vi "extract galvo voltage readout clusterinput (SubVI).vi"(0 "file path (use dialog)":path=path "F:/20220627-135231calib/waveforms.pico", 5 "cluster":T1={"# of avg for single waveform"=0, "skip [us]"=0.0, "Nzf*Nv"=0, "ofst"=0.0, "# of avg for volumes"=0, "limit data length"=FALSE, "num of frames"=7500, "Nv"=7500}) -> (3 "element":dbl=5713585.0 format="%#.6g", 4 "sampling period [s]":dbl=2.0000000000000002e-07, 6 "img scan tangent":dbl[][](array[numeric]), 8 "path":path=path "F:/20220627-135231calib/waveforms.pico", 10 "img scan voltage":dbl[][](array[numeric]), 14 "img scan monitor":dbl[][](array[numeric])=[[17426.8575, 17426.57890625, 17426.393014705885, 17426.015972222223, 17426.046052631584, 17426.081875000003, 17426.223214285717, 17426.462215909094, 17426.573641304352, 17426.58333333334, 17426.650000000005, 17426.70192307693, 17426.684259259262, 17426.62790178572, 17426.683405172418, 17426.428541666668, 17426.769583333335, 17426.764791666665, 17426.585000000003, 17426.678541666668, 17426.580208333336, 17426.766041666666, 17426.400833333333, 17425.925, 17425.767708333333, 17425.599374999998, 17425.643958333334, 17425.721875, 17425.934791666667, 17426.01666666667, 17405.65229166667, 17385.227916666667, 17364.631458333337, 17344.195208333334, 17323.627500000002, 17302.979375000003, 17282.143333333333, 17261.662708333333, 17240.9425, 17220.465208333335, 17199.550833333335, 17178.76104166667, 17158.0975, 17137.55375, 17116.852916666667, 17096.455416666668, 17075.99979166667, 17055.875000000004, 17035.641458333335, 17015.165, 16994.666875000003, 16973.95625, 16953.879375, 16933.634791666667, 16913.513333333332, 16893.22625, 16872.86166666667, 16852.333125, 16831.65479166667, 16811.39875, 16811.619166666667, 16811.996875, 16812.30375, 16812.505833333336, 16812.805, 16813.115416666664, 16813.765208333334, 16813.975416666668, 16814.656250000004, 16814.768333333333, 16815.377291666668, 16815.921875, 16816.422708333335, 16816.803333333337, 16817.303958333338, 16817.65104166667, 16817.842708333334, 16817.864375, 16818.0175, 16817.942708333336, 16818.408958333333, 16823.041666666668, 16827.319791666665, 16831.751458333332, 16836.23916666667, 16840.49166666667, 16844.815833333334, 16849.262708333335, 16853.55625, 16858.025208333333, 16862.329375, 16866.619583333333, 16871.013541666667, 16875.337708333336, 16879.691458333335, 16884.1675, 16888.345625, 16892.422083333335, 16896.401875, 16900.792083333337, 16905.074583333335, 16909.230625, 16913.635833333334, 16918.071875, 16922.290833333333, 16926.32729166667, 16930.582708333335, 16934.843333333334, 16939.024791666667, 16943.72604166667, 16947.92625, 16947.920000000002, 16948.140625000004, 16948.402916666666, 16948.552708333336, 16948.504375, 16948.75104166667, 16948.672083333335, 16948.811250000002, 16948.748541666668, 16948.98083333333, 16949.103541666667, 16949.432500000003, 16949.969166666666, 16949.946041666666, 16950.256666666668, 16950.129166666666, 16950.352916666667, 16950.579791666667, 16950.901458333334, 16951.132916666666, 16951.583541666667, 16951.837291666667, 16951.97125, 16952.314375, 16952.725208333333, 16953.061875, 16953.691875, 16954.147916666665, 16954.536666666667, 16954.955625, 16955.362083333333, 16955.455625, 16955.776666666665, 16955.82875, 16956.381875, 16956.631250000002, 16956.922083333335, 16957.26166666667, 16957.630416666667, 16957.507291666665, 16957.776041666668, 16957.779791666668, 16957.724583333336, 16957.912291666664, 16957.810833333333, 16958.213958333334, 16958.580416666668, 16958.618125, 16958.52, 16958.594583333335, 16958.387291666666, 16958.096041666668, 16957.90145833333, 16957.857083333332, 16957.859791666666, 16957.609375, 16957.483750000003, 16957.221875000003, 16956.683333333334, 16956.31645833333, 16955.692291666666, 16955.479583333334, 16955.1125, 16954.97, 16954.416875000003, 16954.218958333335, 16953.786458333336, 16953.43041666667, 16952.913125000003, 16952.55479166667, 16952.136875, 16951.79291666667, 16955.91, 16959.946875, 16963.795416666668, 16967.703541666666, 16971.37895833333, 16975.24208333333, 16979.29583333333, 16983.233749999996, 16987.069999999996, 16991.212916666664, 16995.311666666665, 16999.31645833333, 17003.39270833333, 17007.47979166666, 17011.363958333328, 17015.54895833333, 17019.71833333333, 17023.537291666664, 17027.80083333333, 17031.81333333333, 17035.665625, 17039.81625, 17044.251458333332, 17048.425, 17052.4475, 17056.288333333334, 17060.481875, 17064.758541666666, 17068.954166666666, 17072.884375, 17072.548333333332, 17072.505, 17072.415625, 17072.205833333333, 17072.14291666667, 17072.242916666666, 17072.09479166667, 17071.799375000002, 17071.773750000004, 17071.26604166667, 17070.87666666667, 17070.459583333337, 17070.280833333338, 17070.02229166667, 17069.533958333333, 17069.177291666667, 17068.915, 17069.008541666666, 17068.623125, 17068.477499999997, 17068.51916666666, 17068.037499999995, 17067.816249999996, 17067.35208333333, 17067.600208333333, 17067.69125, 17067.655208333334, 17067.527916666666, 17067.34375, 17067.466875000002, 17067.292291666665, 17067.10166666667, 17066.90666666667, 17066.855208333334, 17066.418541666666, 17066.206250000003, 17066.17541666667, 17066.291458333333, 17066.33520833333, 17066.49583333333, 17066.335, 17066.270833333332, 17066.285625, 17066.708541666667, 17066.894791666666, 17067.071458333336, 17067.162500000002, 17067.053541666668, 17067.199375000004, 17067.29666666667, 17067.26229166667, 17067.362708333338, 17067.22979166667, 17067.215833333335, 17067.005, 17066.970208333336, 17066.72354166667, 17066.776458333337, 17066.567916666667, 17066.789375, 17066.758125, 17066.709583333333, 17066.37, 17066.189791666668, 17066.421041666665, 17066.268125, 17066.104166666668, 17065.90645833333, 17065.65270833333, 17065.312916666666, 17065.384583333336, 17067.836874999997, 17071.816875, 17075.64375, 17079.814791666668, 17083.854791666665, 17087.688749999998, 17091.658749999995, 17095.795625, 17099.879166666666, 17103.79645833333, 17108.04520833333, 17112.21895833333, 17116.45604166666, 17120.72166666666, 17124.82145833333, 17128.939166666663, 17132.769791666662, 17136.88458333333, 17140.837499999998, 17145.071041666662, 17149.218541666665, 17153.565, 17157.84020833333, 17162.007291666665, 17165.927083333332, 17170.08208333333, 17174.406041666665, 17178.722916666666, 17183.076666666664, 17187.449166666665, 17189.39520833333, 17189.391041666666, 17189.241666666665, 17189.335208333334, 17189.053958333334, 17189.375, 17189.44854166667, 17189.32541666667, 17189.19541666667, 17189.30666666667, 17189.25875, 17189.172708333335, 17189.151250000003, 17188.863125, 17188.919375000005, 17188.666250000002, 17188.68854166667, 17188.908750000006, 17188.71541666667, 17188.712916666675, 17188.64229166667, 17189.000625, 17189.03104166667, 17189.037916666668, 17189.397708333334, 17189.065, 17188.76916666667, 17188.645208333335, 17188.52166666667, 17188.66791666667, 17188.525833333333, 17188.623541666668, 17188.731875, 17188.72395833333, 17188.74395833333, 17188.216875, 17188.180416666662, 17188.01583333333, 17187.985624999998, 17187.840416666666, 17187.9075, 17187.936458333334, 17187.71958333333, 17187.809583333332, 17187.68645833333, 17188.006666666664, 17188.085625, 17187.90270833333, 17187.715625, 17187.607291666667, 17187.539583333335, 17187.312499999996, 17187.372291666663, 17187.349999999995, 17187.29395833333, 17187.52229166666, 17187.730416666665, 17187.824166666665, 17187.821041666666, 17187.667499999996, 17187.27583333333, 17187.174791666665, 17187.104166666664, 17186.55895833333, 17186.507291666665, 17186.649166666666, 17186.443958333333, 17186.470833333336, 17186.299375000006, 17186.303541666668, 17186.120208333337, 17185.978958333337, 17189.871666666666, 17193.96625, 17198.127500000002, 17202.263541666667, 17206.455208333336, 17210.33229166667, 17214.595, 17218.28895833333, 17222.518958333334, 17226.473958333332, 17230.407291666663, 17234.408124999998, 17238.576874999995, 17242.83166666666, 17247.050624999996, 17251.144791666662, 17255.35833333333, 17259.321874999994, 17263.672916666663, 17267.643541666665, 17271.743749999998, 17276.409791666665, 17280.880833333333, 17285.181458333333, 17289.435416666664, 17293.804791666666, 17298.1225, 17302.303125, 17306.237291666668, 17310.470208333332, 17311.01625, 17311.168125, 17311.376875, 17311.425208333334, 17311.447708333337, 17311.601458333334, 17311.787916666668, 17312.389375000002, 17312.217500000002, 17312.434375, 17312.505416666667, 17312.490416666667, 17312.340625, 17312.19916666667, 17312.161458333336, 17312.093958333335, 17312.44916666667, 17312.553541666668, 17312.748958333334, 17312.909583333334, 17313.022708333334, 17313.220416666667, 17313.186458333334, 17313.358541666665, 17313.411249999997, 17313.367916666666, 17313.41020833333, 17313.264583333334, 17313.798958333333, 17313.68354166667, 17313.428750000003, 17313.378333333334, 17313.289583333335, 17313.281250000004, 17313.363125, 17313.63125, 17313.602083333335, 17313.453333333335, 17314.02104166667, 17314.069791666672, 17314.462083333336, 17314.58291666667, 17314.642708333336, 17314.706458333338, 17314.6025, 17314.71479166667, 17314.408541666668, 17314.442083333335, 17314.090416666666, 17314.10583333333, 17313.910833333335, 17313.652916666666, 17313.76125, 17313.76125, 17313.832291666666, 17313.872708333332, 17313.939583333333, 17314.49895833333, 17314.488125, 17314.895, 17314.988541666666, 17315.07625, 17315.161874999998, 17315.241666666665, 17315.106666666667, 17315.085625, 17315.241458333334, 17315.402083333334, 17315.289375, 17315.393125, 17315.255833333333, 17315.314583333333, 17319.186666666665, 17323.182291666664, 17327.20270833333, 17331.295416666664, 17335.578124999996, 17339.690624999996, 17344.006041666664, 17347.847916666662, 17351.89395833333, 17355.687499999993, 17359.47333333333, 17363.35708333333, 17367.400625, 17371.44395833333, 17375.41958333333, 17379.094791666666, 17382.835624999996, 17386.513541666664, 17390.534375, 17394.35833333333, 17398.18520833333, 17402.037916666664, 17405.970624999998, 17409.86770833333, 17413.515624999996, 17417.491874999996, 17421.06520833333, 17424.766666666666, 17428.231041666666, 17431.965416666666, 17432.111249999998, 17432.184999999998, 17431.99833333333, 17431.703124999996, 17431.38875, 17430.977291666666, 17430.809166666666, 17431.025416666667, 17430.968333333334, 17431.06604166667, 17430.951041666667, 17430.79375, 17430.682708333334, 17430.123333333333, 17430.102083333335, 17429.75375, 17429.783958333333, 17429.540833333336, 17429.470416666667, 17429.403333333335, 17429.46416666667, 17429.374375, 17429.14625, 17429.01291666667, 17429.031875, 17428.852916666667, 17429.01354166667, 17429.01291666667, 17429.211458333335, 17429.173333333336, 17428.757500000003, 17428.788750000003, 17428.864583333336, 17428.865625000002, 17428.74229166667, 17428.798958333336, 17428.766250000004, 17428.61354166667, 17428.497916666667, 17428.079791666667, 17428.09416666667, 17428.026250000003, 17427.98895833334, 17428.287083333336, 17428.118333333336, 17428.312500000004, 17428.13291666667, 17428.297291666666, 17428.23, 17428.439166666667, 17428.378125000003, 17428.420208333337, 17428.55791666667, 17428.456458333338, 17428.284375000003, 17428.17979166667, 17428.19125, 17428.396875000002, 17428.14666666667, 17428.166250000002, 17428.00625, 17427.863125, 17428.001041666666, 17427.99229166667, 17427.888125, 17427.913125, 17427.857083333332, 17427.8125, 17427.89375, 17428.12104166667, 17427.867291666666, 17428.255624999998, 17432.389791666665, 17436.71958333333, 17441.075208333332, 17445.435, 17449.697083333333, 17453.75270833333, 17458.295, 17462.460208333334, 17466.614791666667, 17471.070625, 17475.374583333334, 17479.895625, 17484.156875, 17488.39625, 17492.415, 17496.401250000003, 17500.887291666666, 17504.940416666668, 17509.587291666667, 17513.759166666667, 17518.013958333333, 17522.553750000003, 17527.107916666668, 17531.75479166667, 17536.162500000002, 17540.570625, 17544.990416666667, 17549.476666666666, 17554.101041666665, 17558.422916666663, 17558.953333333327, 17559.28083333333, 17559.575833333325, 17559.61604166666, 17559.911041666663, 17560.37895833333, 17560.30375, 17560.497499999998, 17560.67645833333, 17560.788541666665, 17561.008749999997, 17561.085833333334, 17561.520208333335, 17561.868125, 17562.010208333337, 17562.339375, 17562.324166666665, 17562.667708333334, 17563.001250000005, 17563.405208333337, 17563.263125, 17563.37875, 17563.527500000004, 17563.232500000002, 17563.45354166667, 17563.625000000004, 17563.801250000004, 17564.04729166667, 17564.189583333336, 17564.31645833334, 17564.499583333338, 17564.479375000003, 17564.27395833334, 17564.484375000004, 17564.61479166667, 17564.93145833334, 17565.070416666673, 17565.194791666676, 17565.54291666667, 17565.52395833334, 17565.83375, 17566.275, 17566.440208333333, 17566.596875, 17567.001041666666, 17567.242916666666, 17567.837083333336, 17568.307708333337, 17568.490208333336, 17568.415416666667, 17568.878541666665, 17569.045624999995, 17569.22958333333, 17569.927083333332, 17570.251875, 17570.685416666667, 17571.07625, 17571.371875, 17571.741250000003, 17571.689583333333, 17571.573333333337, 17571.56791666667, 17571.967708333334, 17571.813541666666, 17571.82458333333, 17572.045416666664, 17572.501666666663, 17572.698958333334, 17572.720208333332, 17572.939583333333, 17572.947083333333, 17572.588333333333, 17576.981875, 17581.562916666666, 17586.169375, 17590.86625, 17595.529375, 17600.363125, 17605.247291666667, 17610.116875, 17614.657291666666, 17619.321666666667, 17624.047291666666, 17628.570208333334, 17633.326666666668, 17637.698750000003, 17642.445000000003, 17646.612083333337, 17650.999791666673, 17655.749791666673, 17660.43583333334, 17665.46979166667, 17669.975833333338, 17675.01645833334, 17679.93104166667, 17684.220625000005, 17688.696250000005, 17693.11270833334, 17697.73520833334, 17702.44041666667, 17707.286666666674, 17712.382708333338, 17712.762916666674, 17713.058125000003, 17712.991250000006, 17712.968750000004, 17712.905000000006, 17712.69666666667, 17712.778541666667, 17712.751458333332, 17712.941666666666, 17713.056875, 17713.289374999997, 17713.363124999996, 17713.23208333333, 17713.563749999994, 17713.26895833333, 17713.937291666665, 17714.15208333333, 17714.207499999997, 17714.41770833333, 17714.420624999995, 17714.625833333335, 17714.47666666667, 17714.431666666667, 17714.47333333333, 17714.320625, 17714.757291666665, 17714.89916666667, 17715.175833333335, 17715.108125000002, 17715.015208333334, 17715.25770833333, 17715.310416666667, 17715.355, 17715.310208333332, 17715.493333333336, 17715.92270833333, 17715.953749999997, 17716.279375, 17716.343125000003, 17716.49208333333, 17716.622916666667, 17716.638541666667, 17716.616041666664, 17716.605416666665, 17716.791666666668, 17716.646041666667, 17716.635000000002, 17716.948125000003, 17716.783541666668, 17716.94541666667, 17717.165833333333, 17717.494791666668, 17717.81229166667, 17718.192708333332, 17718.565000000002, 17718.460833333334, 17718.483125000002, 17718.345416666667, 17718.59979166667, 17718.823750000003, 17718.906666666673, 17718.939166666667, 17719.302083333336, 17719.661458333336, 17719.930833333336, 17719.830208333333, 17719.600833333334, 17719.541041666667, 17719.756875000003, 17719.843125000003, 17719.809166666666, 17720.06270833333, 17724.825624999998, 17729.234166666665, 17733.76145833333, 17738.269791666662, 17742.832291666666, 17747.098749999997, 17751.614791666667, 17756.153333333332, 17760.655833333334, 17765.231875, 17769.673333333336, 17774.309583333335, 17778.711250000004, 17783.642708333336, 17788.178541666668, 17792.519375, 17796.949166666673, 17801.35729166667, 17805.989583333336, 17810.56333333334, 17814.98625, 17819.51291666667, 17824.12916666667, 17828.89604166667, 17833.700833333332, 17838.32125, 17842.66645833333, 17847.205625, 17851.826041666667, 17856.424375000002, 17856.584583333337, 17856.662708333337, 17856.90166666667, 17856.827083333334, 17857.083749999998, 17857.457083333335, 17857.621875, 17857.640625, 17857.584166666667, 17857.568958333337, 17857.744583333337, 17857.87166666667, 17858.274583333336, 17858.11416666667, 17858.420416666668, 17858.851875000004, 17858.96875, 17859.286875, 17859.548958333333, 17859.865625, 17860.187083333334, 17860.258958333332, 17860.147500000003, 17859.74375, 17859.915, 17859.844374999997, 17860.125625, 17860.349583333333, 17860.196875, 17860.269166666665, 17860.153958333332, 17860.212916666667, 17860.27375, 17860.45291666667, 17860.591666666667, 17860.347708333335, 17860.5825, 17860.496041666665, 17860.421458333334, 17860.421041666665, 17860.177708333333, 17860.106875, 17859.785, 17859.662083333336, 17859.467916666665, 17859.39875, 17859.54416666667, 17859.34291666667, 17859.193125, 17859.215833333335, 17858.99104166667, 17859.028125000004, 17858.901250000003, 17859.311458333337, 17859.363750000004, 17859.553958333338, 17859.84125, 17859.70604166667, 17859.92583333334, 17859.525416666664, 17859.675, 17859.806458333333, 17859.809166666666, 17859.828125, 17859.693541666667, 17859.997708333332, 17859.88625, 17860.01354166667, 17860.36125, 17860.511458333338, 17860.583125, 17860.698958333334, 17865.431041666667, 17870.288541666665, 17875.00479166667, 17879.683333333338, 17884.015, 17888.80479166667, 17893.244375, 17897.69854166667, 17902.440833333338, 17906.903125000004, 17911.544583333332, 17915.793958333332, 17920.141666666666, 17924.671875, 17928.87958333333, 17933.14083333333, 17937.52895833333, 17942.353333333333, 17946.830208333333, 17951.482083333332, 17956.046458333334, 17960.680208333335, 17965.243958333336, 17969.855208333334, 17974.847083333338, 17979.428750000003, 17983.692708333332, 17988.02375, 17992.522916666665, 17997.026250000003, 17997.093125, 17996.831875, 17996.775625, 17996.596666666665, 17996.466666666667, 17996.358333333334, 17996.470833333333, 17996.575624999998, 17996.736875, 17996.97645833333, 17997.234166666665, 17997.649999999998, 17997.883958333332, 17997.76375, 17997.904999999995, 17998.27895833333, 17998.6675, 17999.070625, 17999.23125, 17999.447708333333, 17999.5025, 17999.65604166667, 17999.931875, 17999.961874999997, 17999.733750000003, 17999.748541666668, 17999.99125, 18000.41270833333, 18000.90583333333, 18001.290416666663, 18001.52583333333, 18001.932083333326, 18002.133749999994, 18002.454374999994, 18003.04833333333, 18003.079999999994, 18003.128958333327, 18003.02083333333, 18002.841249999994, 18002.866874999996, 18002.963749999995, 18002.959791666664, 18002.91895833333, 18003.259791666664, 18003.276041666668, 18003.167291666665, 18003.002083333333, 18002.946249999997, 18003.148125, 18003.074375, 18003.123333333333, 18003.216666666667, 18002.94020833333, 18003.022291666664, 18002.952291666665, 18003.008541666666, 18003.28125, 18003.285416666666, 18003.064374999998, 18002.5, 18002.284166666665, 18002.10916666667, 18002.086666666666, 18002.347708333335, 18002.294583333332, 18002.263541666667, 18002.196458333336, 18002.32354166667, 18002.4425, 18002.299583333333, 18002.119583333333, 18002.101041666665, 18006.778125, 18011.66416666667, 18016.434166666666, 18021.279375, 18025.890833333335, 18030.50791666667, 18034.964583333334, 18039.574375, 18044.35958333333, 18048.9625, 18053.977291666666, 18058.55416666666, 18063.43291666667, 18068.2075, 18072.51479166667, 18076.949791666666, 18081.306458333333, 18086.092499999995, 18090.710000000003, 18095.080416666668, 18099.795625000002, 18103.931875000002, 18108.39520833333, 18113.027291666665, 18117.621666666666, 18122.022916666665, 18126.535625, 18131.090624999997, 18135.36583333333, 18139.604374999995, 18139.604166666668, 18139.129375, 18138.74083333333, 18138.38583333333, 18138.261875, 18137.772708333334, 18137.496458333335, 18137.260208333333, 18136.80020833333, 18136.661666666667, 18136.126666666667, 18135.71958333333, 18135.490624999995, 18135.203125, 18135.113749999997, 18134.811041666664, 18134.919999999995, 18134.941666666666, 18134.667916666665, 18134.74979166667, 18134.413541666665, 18134.48041666667, 18134.227291666666, 18134.145000000004, 18134.40666666667, 18134.423958333333, 18134.30104166667, 18134.21125, 18134.185000000005, 18134.41416666667, 18133.943750000002, 18133.94791666667, 18134.015208333334, 18134.026041666668, 18134.13375, 18134.115416666667, 18134.052708333333, 18133.76208333333, 18133.699375, 18133.494166666664, 18133.369999999995, 18133.380416666663, 18132.876041666666, 18132.692499999997, 18132.640624999996, 18132.595625, 18132.587916666667, 18132.471875000003, 18132.786458333336, 18132.454791666663, 18132.319791666665, 18132.17479166667, 18132.103541666667, 18131.938749999998, 18131.14333333333, 18130.853125, 18130.718125, 18130.646666666667, 18130.534166666668, 18130.134374999998, 18130.0525, 18129.869166666667, 18129.57354166667, 18129.614166666663, 18129.43895833333, 18129.711666666666, 18129.736458333333, 18129.997291666667, 18130.105208333334, 18129.974583333333, 18129.94833333333, 18129.91833333333, 18134.302499999998, 18138.29395833333, 18142.307291666664, 18146.33583333333, 18150.07333333333, 18153.919791666664, 18157.783958333326, 18161.89458333333, 18166.15083333333, 18169.884374999998, 18173.823749999996, 18177.920833333334, 18182.038749999996, 18186.059166666662, 18190.163749999996, 18194.44020833333, 18198.520624999997, 18202.647083333333, 18206.731875, 18210.69, 18214.860625000005, 18218.65479166667, 18222.64291666667, 18226.339375000003, 18230.301875, 18234.059166666666, 18238.032500000005, 18242.061666666665, 18246.36729166667, 18250.29916666667, 18250.445, 18250.452291666665, 18250.389583333334, 18250.647500000003, 18250.80458333333, 18251.025416666664, 18250.939166666667, 18251.092083333333, 18251.015, 18251.351041666665, 18251.33958333333, 18251.237708333338, 18251.470208333336, 18251.51291666667, 18251.688125000004, 18251.75791666667, 18251.855, 18252.112708333334, 18252.575833333332, 18252.911458333332, 18253.490833333333, 18253.78583333333, 18254.137291666662, 18254.439583333333, 18254.89145833333, 18255.257916666666, 18255.272916666665, 18255.690624999996, 18256.016458333328, 18256.666666666664, 18256.804583333327, 18257.15541666666, 18257.210833333327, 18257.195833333328, 18257.468958333327, 18257.19270833333, 18257.39833333333, 18257.779374999995, 18257.73020833333, 18257.756874999995, 18258.02666666666, 18258.22895833333, 18258.438124999993, 18258.754374999997, 18258.791875, 18258.705208333333, 18258.972844827582, 18259.034151785716, 18258.975694444445, 18258.93918269231, 18258.599000000002, 18258.71640625, 18258.53097826087, 18258.477556818183, 18258.199702380953, 18258.251875, 18258.570065789478, 18258.438194444447, 18258.09191176471, 18257.521484375004], [17417.01875, 17419.06875, 17427.35, 17425.64375, 17428.1375, 17430.8125, 17432.91875, 17435.54375, 17422.5375, 17430.26875, 17423.8625, 17430.71875, 17430.25, 17421.73125, 17427.0, 17422.4, 17423.41875, 17419.60625, 17426.5875, 17426.7625, 17429.05, 17431.48125, 17429.025, 17426.80625, 17428.25, 17428.0, 17426.225, 17425.10625, 17428.2375, 17419.0375, 17427.25, 17418.925, 17421.95625, 17428.45, 17425.1875, 17436.3875, 17421.9625, 17421.26875, 17417.81875, 17425.21875, 17425.2, 17433.05625, 17436.6375, 17424.1875, 16816.06875, 16809.66875, 16805.525, 16806.51875, 16809.55625, 16807.31875, 16803.96875, 16817.0625, 16807.41875, 16812.4875, 16800.81875, 16804.30625, 16806.31875, 16808.79375, 16807.2125, 16807.1125, 16813.58125, 16815.18125, 16814.95, 16814.15625, 16810.24375, 16815.06875, 16819.65625, 16813.93125, 16814.175, 16816.60625, 16814.2625, 16817.2, 16816.2875, 16816.50625, 16822.68125, 16821.0, 16814.73125, 16812.58125, 16818.53125, 16816.63125, 16823.4625, 16823.36875, 16827.84375, 16815.85, 16819.0875, 16820.64375, 16821.34375, 16820.2125, 16822.23125, 16817.525, 16819.33125, 16815.83125, 16819.54375, 16811.9125, 16824.23125, 16954.05, 16948.0, 16946.88125, 16948.80625, 16944.18125, 16943.9875, 16950.60625, 16945.09375, 16950.575, 16951.80625, 16949.70625, 16946.55, 16942.30625, 16949.14375, 16950.9125, 16948.80625, 16945.6625, 16947.2375, 16947.55625, 16947.5625, 16945.325, 16953.5, 16953.29375, 16948.8, 16938.61875, 16946.99375, 16943.65, 16944.9875, 16952.95, 16950.2375, 16953.8625, 16954.61875, 16954.75, 16953.3, 16942.73125, 16951.3875, 16948.2375, 16949.26875, 16948.69375, 16958.775, 16953.3875, 16956.41875, 16958.40625, 16948.45, 16960.23125, 16944.98125, 16952.375, 16954.04375, 16957.20625, 16954.50625, 16958.84375, 16961.1125, 16957.3125, 16959.09375, 16950.94375, 16957.09375, 16962.55, 16958.66875, 16964.6125, 16962.80625, 16966.05625, 16957.425, 16964.38125, 16954.8625, 16959.325, 16958.86875, 16956.9625, 16959.45625, 16959.75625, 16955.08125, 16961.45, 16956.53125, 16956.75, 16954.08125, 16957.1875, 16957.075, 16963.36875, 16955.175, 16954.2625, 16956.74375, 16952.625, 16952.375, 16951.475, 16957.7625, 16951.025, 16949.58125, 16958.78125, 16950.8125, 16948.45625, 16951.8, 16947.33125, 16951.04375, 16953.36875, 16950.5875, 16942.73125, 16952.93125, 16943.9875, 16948.775, 16944.2375, 16944.33125, 16948.9125, 16946.2125, 17080.2625, 17075.1875, 17072.64375, 17074.31875, 17073.63125, 17071.06875, 17075.875, 17074.88125, 17067.7125, 17076.6625, 17074.4375, 17077.90625, 17073.3125, 17072.19375, 17075.30625, 17076.3625, 17073.5375, 17066.36875, 17075.2375, 17071.41875, 17068.9375, 17075.10625, 17075.7875, 17078.1375, 17064.6625, 17064.0, 17070.04375, 17072.63125, 17074.78125, 17064.11875, 17070.18125, 17073.8875, 17069.9625, 17068.025, 17071.74375, 17074.06875, 17071.43125, 17066.01875, 17066.94375, 17061.43125, 17062.75625, 17065.39375, 17067.95, 17064.4375, 17060.65625, 17065.6625, 17065.66875, 17069.175, 17063.675, 17067.05, 17070.1875, 17060.65625, 17069.15, 17064.2125, 17072.10625, 17066.73125, 17068.9625, 17068.8125, 17069.25625, 17067.8125, 17064.94375, 17068.16875, 17064.1125, 17066.48125, 17058.64375, 17067.7, 17070.50625, 17069.5, 17068.25625, 17066.25, 17057.93125, 17063.46875, 17068.39375, 17077.125, 17066.24375, 17070.9625, 17068.4, 17065.90625, 17068.05, 17069.96875, 17069.15625, 17063.66875, 17065.1625, 17063.79375, 17065.78125, 17065.6875, 17061.5625, 17070.4, 17063.0, 17074.45625, 17064.00625, 17066.7125, 17053.925, 17061.075, 17065.58125, 17063.1125, 17065.5875, 17063.56875, 17060.64375, 17056.05625, 17060.08125, 17137.0375, 17187.79375, 17191.93125, 17191.375, 17192.1625, 17183.41875, 17185.00625, 17192.15625, 17192.475, 17186.675, 17191.13125, 17190.375, 17190.90625, 17193.75, 17188.68125, 17185.09375, 17185.31875, 17186.44375, 17193.04375, 17191.0125, 17191.1375, 17184.31875, 17189.33125, 17190.59375, 17180.70625, 17190.2375, 17193.2875, 17190.15, 17186.66875, 17191.25625, 17195.41875, 17187.66875, 17187.45, 17194.18125, 17183.725, 17193.05, 17187.2125, 17188.4625, 17188.575, 17190.0125, 17189.69375, 17187.79375, 17190.2625, 17185.10625, 17190.36875, 17177.5, 17185.9875, 17193.05, 17187.24375, 17190.9375, 17189.01875, 17195.06875, 17190.24375, 17190.8, 17191.5, 17180.25625, 17184.4125, 17186.43125, 17182.9625, 17195.64375, 17191.15625, 17190.6, 17190.7, 17193.94375, 17184.325, 17177.2375, 17186.11875, 17183.525, 17187.66875, 17185.65625, 17191.70625, 17188.6625, 17183.75625, 17187.80625, 17186.675, 17187.10625, 17188.35625, 17187.5625, 17181.63125, 17187.6875, 17186.9875, 17188.25625, 17192.0375, 17190.13125, 17189.81875, 17187.10625, 17190.65625, 17189.24375, 17182.86875, 17191.0375, 17179.40625, 17187.56875, 17188.58125, 17177.5875, 17182.775, 17181.49375, 17179.9625, 17184.33125, 17182.525, 17185.78125, 17186.20625, 17184.425, 17300.5375, 17310.64375, 17311.5125, 17311.1875, 17314.10625, 17303.875, 17309.5125, 17298.50625, 17313.8875, 17306.90625, 17310.0375, 17310.15625, 17314.88125, 17314.75, 17317.225, 17312.06875, 17309.275, 17309.94375, 17309.9375, 17306.6875, 17311.5875, 17317.56875, 17316.90625, 17310.5125, 17307.58125, 17315.4125, 17312.05625, 17311.2, 17304.23125, 17311.4125, 17316.91875, 17315.2, 17317.775, 17312.6375, 17314.78125, 17308.4875, 17315.10625, 17316.55, 17308.73125, 17313.4125, 17312.16875, 17309.70625, 17310.3875, 17310.50625, 17316.09375, 17310.04375, 17319.93125, 17313.075, 17315.8, 17311.50625, 17314.98125, 17323.5, 17315.8875, 17315.675, 17309.1625, 17314.1125, 17313.325, 17306.83125, 17320.2625, 17307.95, 17309.275, 17313.6875, 17315.1125, 17312.3875, 17317.2375, 17316.53125, 17314.23125, 17312.0875, 17325.7625, 17314.875, 17323.9375, 17313.33125, 17312.18125, 17312.41875, 17312.975, 17313.4125, 17310.74375, 17314.08125, 17305.25, 17311.96875, 17309.13125, 17315.7625, 17319.1375, 17315.675, 17311.29375, 17315.325, 17315.33125, 17323.6125, 17319.9375, 17320.15625, 17312.08125, 17316.31875, 17317.68125, 17314.78125, 17313.1875, 17315.9, 17318.90625, 17316.90625, 17322.38125, 17317.9875, 17319.81875, 17315.09375, 17428.34375, 17432.2875, 17433.5875, 17436.19375, 17439.225, 17437.45625, 17434.7125, 17427.225, 17430.5125, 17429.56875, 17432.7125, 17432.1875, 17432.6, 17436.625, 17434.6, 17433.86875, 17432.1625, 17430.49375, 17432.70625, 17431.0375, 17432.4875, 17430.3625, 17431.16875, 17432.8125, 17428.34375, 17436.19375, 17429.58125, 17429.03125, 17423.75, 17427.125, 17432.71875, 17434.5, 17427.9875, 17427.3375, 17429.79375, 17425.1125, 17429.66875, 17433.7125, 17428.8, 17432.5, 17429.2625, 17427.46875, 17429.26875, 17419.84375, 17433.9625, 17423.41875, 17433.06875, 17423.2, 17430.59375, 17429.025, 17434.3125, 17427.66875, 17424.325, 17428.8125, 17428.9125, 17430.825, 17434.4, 17429.0125, 17429.70625, 17425.98125, 17420.24375, 17435.4375, 17430.2625, 17427.36875, 17426.09375, 17426.8125, 17428.6875, 17429.13125, 17425.33125, 17419.95625, 17429.69375, 17425.43125, 17428.15, 17428.7875, 17428.9, 17429.24375, 17427.68125, 17428.13125, 17428.575, 17435.3, 17432.48125, 17428.93125, 17428.45625, 17425.76875, 17423.75, 17427.6875, 17434.74375, 17435.18125, 17422.2, 17426.56875, 17415.44375, 17431.14375, 17434.4, 17427.10625, 17422.96875, 17427.5625, 17427.00625, 17427.79375, 17427.76875, 17426.775, 17422.08125, 17437.08125, 17552.175, 17558.68125, 17559.56875, 17560.0375, 17555.54375, 17549.8, 17564.84375, 17560.25625, 17557.11875, 17562.60625, 17557.575, 17561.4, 17551.5875, 17554.86875, 17555.30625, 17554.76875, 17556.78125, 17548.1625, 17554.85, 17556.3, 17562.04375, 17563.3, 17559.59375, 17566.96875, 17559.2375, 17560.0375, 17560.3625, 17561.3625, 17560.8125, 17566.7375, 17568.0875, 17568.50625, 17568.41875, 17561.24375, 17564.39375, 17563.8375, 17562.5875, 17566.06875, 17562.4875, 17565.96875, 17564.18125, 17563.7125, 17564.61875, 17565.30625, 17559.56875, 17564.64375, 17556.325, 17558.46875, 17564.85625, 17568.41875, 17557.78125, 17566.76875, 17564.05625, 17558.11875, 17565.86875, 17565.18125, 17565.65, 17568.74375, 17565.08125, 17570.54375, 17573.58125, 17567.9, 17562.25625, 17567.55625, 17568.30625, 17573.3375, 17566.75625, 17569.8, 17572.93125, 17565.4, 17573.475, 17576.95, 17569.575, 17570.00625, 17571.69375, 17571.9, 17574.15, 17572.5875, 17570.33125, 17566.175, 17571.675, 17571.78125, 17569.575, 17579.04375, 17575.6125, 17578.1875, 17577.375, 17577.6125, 17576.1625, 17568.99375, 17570.09375, 17567.7375, 17574.25, 17562.93125, 17568.6375, 17579.9625, 17580.44375, 17575.71875, 17573.56875, 17571.98125, 17573.7, 17566.1875, 17701.38125, 17707.4375, 17709.8875, 17712.80625, 17714.04375, 17717.6, 17716.85625, 17712.2625, 17707.8875, 17711.7125, 17711.34375, 17714.73125, 17718.30625, 17709.35, 17719.7625, 17702.625, 17707.79375, 17711.49375, 17710.675, 17718.75625, 17709.43125, 17714.15, 17716.075, 17708.65, 17714.7125, 17708.2125, 17712.24375, 17713.1375, 17719.0875, 17719.06875, 17712.7875, 17716.29375, 17707.88125, 17712.13125, 17712.13125, 17711.35, 17719.3125, 17711.45, 17713.59375, 17715.16875, 17718.31875, 17716.94375, 17714.375, 17719.3, 17710.91875, 17722.675, 17714.2375, 17713.15625, 17716.98125, 17718.84375, 17715.5875, 17709.675, 17714.725, 17709.9, 17710.13125, 17721.3125, 17716.5, 17721.4375, 17717.05625, 17716.28125, 17720.0625, 17717.875, 17709.21875, 17710.7875, 17717.625, 17724.23125, 17720.24375, 17721.21875, 17715.50625, 17719.6375, 17722.24375, 17717.4125, 17713.7, 17718.98125, 17716.50625, 17718.30625, 17713.90625, 17722.55, 17712.04375, 17723.7, 17722.2, 17719.54375, 17724.25, 17721.3125, 17721.3, 17718.1875, 17717.16875, 17717.30625, 17724.6875, 17723.0, 17722.55, 17718.85, 17720.10625, 17721.56875, 17725.70625, 17721.2125, 17713.3625, 17719.425, 17721.98125, 17722.225, 17721.225, 17725.01875, 17856.5875, 17851.2375, 17852.325, 17853.55625, 17850.78125, 17850.54375, 17847.525, 17859.85625, 17857.275, 17856.825, 17857.49375, 17860.4, 17853.35, 17866.13125, 17853.24375, 17847.53125, 17857.58125, 17855.24375, 17861.51875, 17856.0625, 17852.79375, 17857.36875, 17864.19375, 17864.21875, 17857.50625, 17858.0375, 17852.3375, 17858.4, 17859.8375, 17862.96875, 17861.39375, 17853.58125, 17859.49375, 17851.31875, 17858.48125, 17861.74375, 17852.46875, 17860.41875, 17855.58125, 17856.36875, 17862.7625, 17864.2125, 17865.4375, 17861.31875, 17862.43125, 17860.475, 17861.0875, 17864.7875, 17869.38125, 17865.5625, 17862.4375, 17859.525, 17860.85, 17852.10625, 17862.64375, 17855.91875, 17860.775, 17865.11875, 17855.25625, 17865.1375, 17857.9375, 17855.35, 17861.31875, 17856.69375, 17862.64375, 17854.425, 17859.5125, 17857.825, 17853.34375, 17856.35625, 17855.4625, 17862.0875, 17855.78125, 17857.63125, 17856.60625, 17858.4, 17865.45, 17858.75, 17864.8875, 17866.24375, 17855.69375, 17860.6375, 17857.04375, 17864.4125, 17864.2125, 17861.625, 17869.39375, 17861.0625, 17861.85, 17853.125, 17862.425, 17859.29375, 17861.4, 17857.2625, 17858.60625, 17863.55, 17856.16875, 17861.64375, 17863.775, 17860.8625, 17857.6125, 17865.5625, 17997.74375, 18003.35625, 17998.09375, 17998.75625, 17995.4, 18002.44375, 17998.075, 17999.86875, 17997.9625, 17994.50625, 17996.2875, 17991.89375, 17994.64375, 17997.53125, 17995.625, 17988.9, 17993.49375, 17997.85625, 17996.73125, 17998.85, 17998.33125, 17996.275, 17995.51875, 18001.8875, 18005.925, 17999.09375, 17991.69375, 17990.79375, 17992.5875, 18000.6625, 17999.75, 17995.51875, 17996.40625, 17993.3875, 17991.5, 17999.19375, 18001.45, 18003.0125, 18002.8, 18001.69375, 18004.01875, 18004.36875, 18001.6625, 17993.925, 17999.8625, 18000.11875, 18005.15, 18009.95, 18001.55, 18005.34375, 17999.975, 18000.88125, 18003.79375, 18002.7875, 17999.08125, 17999.5375, 17998.975, 18003.4375, 18007.38125, 18012.2, 18006.8125, 18007.70625, 18002.45625, 18003.00625, 18009.31875, 18000.14375, 18002.91875, 17999.76875, 17997.4125, 18002.4625, 18006.925, 18004.25, 18000.4375, 18004.15, 18000.35, 17996.85625, 18000.19375, 18008.275, 18007.60625, 18003.13125, 18001.44375, 18003.68125, 17995.5, 18005.25, 17996.98125, 18001.225, 18007.15625, 18003.5625, 18000.75, 17995.26875, 18000.3375, 18002.45625, 18001.78125, 18010.8375, 18007.725, 17999.2125, 18000.90625, 18003.58125, 18000.98125, 17998.175, 18001.525, 18003.69375, 18140.75, 18150.73125, 18143.45, 18142.2125, 18138.5375, 18146.7875, 18141.30625, 18141.425, 18145.0, 18141.76875, 18145.94375, 18142.55625, 18143.34375, 18144.4625, 18136.375, 18136.6125, 18131.45, 18138.85, 18138.8625, 18133.56875, 18143.2375, 18134.925, 18141.625, 18138.175, 18138.7375, 18135.61875, 18136.3625, 18134.825, 18129.78125, 18130.85, 18140.74375, 18136.4875, 18131.79375, 18131.5625, 18134.81875, 18132.1125, 18133.01875, 18134.3375, 18131.2, 18137.6125, 18129.89375, 18130.34375, 18136.475, 18135.8375, 18133.69375, 18127.53125, 18134.71875, 18139.5, 18130.65, 18136.025, 18133.15, 18136.93125, 18134.03125, 18135.70625, 18146.5875, 18136.1375, 18132.675, 18132.13125, 18128.99375, 18137.725, 18126.63125, 18136.6125, 18133.8125, 18131.8875, 18138.05, 18131.5625, 18131.1375, 18125.61875, 18129.31875, 18131.45625, 18126.16875, 18130.65625, 18121.34375, 18130.33125, 18132.1375, 18126.18125, 18134.4875, 18136.01875, 18140.0875, 18126.075, 18129.1, 18132.58125, 18131.89375, 18130.7625, 18122.725, 18127.43125, 18128.625, 18129.9875, 18125.61875, 18125.73125, 18124.175, 18131.1125, 18124.94375, 18133.10625, 18132.79375, 18139.74375, 18131.88125, 18133.44375, 18132.55625, 18127.5375, 18125.38125, 18129.75625, 18252.86875, 18250.075, 18252.5375, 18247.0375, 18246.6125, 18251.4125, 18256.0125, 18249.39375, 18256.7875, 18244.5875, 18250.075, 18253.675, 18246.2625, 18248.04375, 18251.7625, 18258.28125, 18248.03125, 18249.525, 18246.71875, 18249.85625, 18250.0625, 18246.93125, 18252.4375, 18250.6375, 18250.75625, 18246.1625, 18251.75625, 18248.4125, 18254.55, 18247.7125, 18257.24375, 18250.29375, 18250.65625, 18254.775, 18251.325, 18258.0375, 18253.425, 18253.98125, 18254.475, 18254.66875, 18249.73125, 18250.61875, 18253.2375, 18249.325, 18257.01875, 18260.375, 18250.94375, 18257.25625, 18260.6125, 18259.925, 18267.44375, 18255.78125, 18262.98125, 18259.70625, 18264.3125, 18257.15625, 18252.20625, 18260.94375, 18264.325, 18267.21875, 18261.38125, 18260.81875, 18252.31875, 18254.325, 18259.51875, 18249.75, 18259.59375, 18265.4125, 18253.0, 18255.46875, 18257.825, 18256.6875, 18259.5125, 18258.8125, 18258.14375, 18257.775]], 15 "img scan":dbl[][](graph))   [LabVIEW 2024]
uses:
  <vilib>/Analysis/baseanly.llb/Mean (DBL).vi
  <vilib>/Analysis/NI_AALBase.lvlib
  <vilib>/Analysis/NI_AALPro.lvlib
panel:
  out "img scan 3":dbl[](graph)
  out "Array 3":i32[](array[numeric])
  out "img scan 2":dbl[](graph)
  out "Array":dbl[](array[numeric])
  out "Numeric 2":i32
  out "Numeric":i32
  in  "analysis unit [s]":dbl=30.0
  out "error out":errorcluster
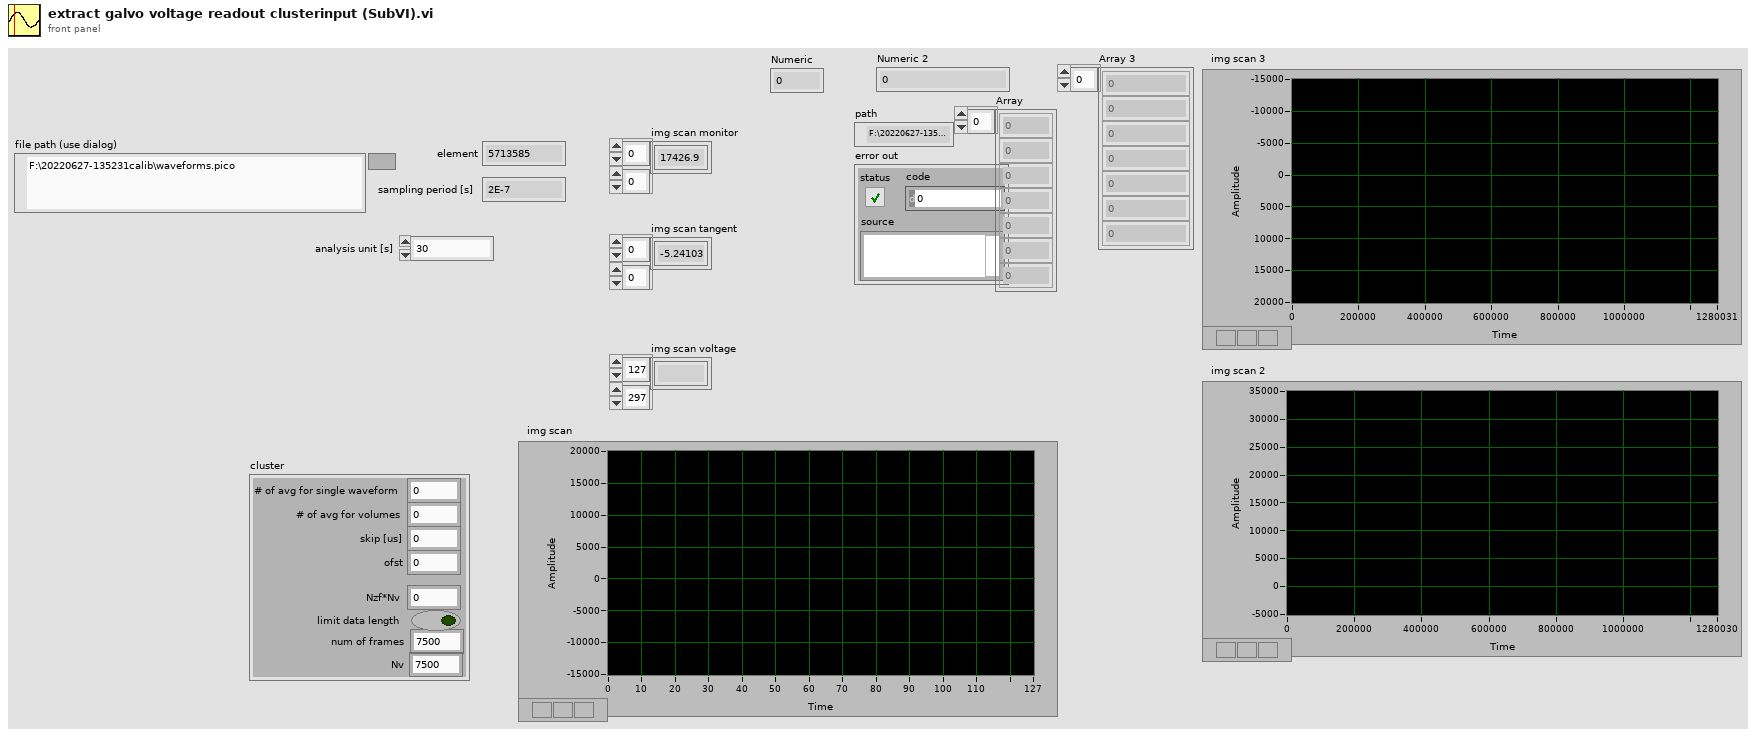
[diagram p1: front panel]
types:
  T1 = cluster{"# of avg for single waveform":u16, "skip [us]":dbl, "Nzf*Nv":i32, "ofst":dbl, "# of avg for volumes":u16, "limit data length":bool, "num of frames":i32, "Nv":i32}
  T2 = cluster{"Channel settings":cluster{"Ch D  sync":cluster{"Enabled":bool, "Coupling":i16, "Range":u16, "Offset":sgl}, "Ch C AWG ":cluster{"Enabled":bool, "Coupling":i16, "Range":u16, "Offset":sgl}, "Ch G scape":cluster{"Enabled":bool, "Coupling":i16, "Range":u16, " Offset":sgl}, "Ch H img scan":cluster{"Enabled":bool, "Coupling":i16, "Range":u16, "Offset":sgl}, "Ch B Cam":cluster{"Enabled":bool, "Coupling":i16, "Range":u16, "Offset":sgl}, "Ch A":cluster{"Enabled":bool, "Coupling":i16, "Range":u16, "Offset":sgl}, "Ch E":cluster{"Enabled":bool, "Coupling":i16, "Range":u16, "Offset":sgl}, "Ch F":cluster{"Enabled":bool, "Coupling":i16, "Range":u16, "Offset":sgl}}, "Acquisition Settings":cluster{"Auto Stop":bool, "Desired Sample Interval":u32, "Pre-trigger Samples":u32, "Post-trigger Samples":u32, "Down-Sample Ratio":u32, "Down-Sample Mode":i32, "Overview Buffer Size":u32, "Time Units":u32}, "Trigger Settings":cluster{"Trigger Enabled":bool, "Trigger Source":enum16{"Channel A", "Channel B", "Channel C", "Channel D", "Channel E", "Channel F", "Channel G", "Channel H"}, "Trig Thresh (16-bit counts)":i16, "Trigger Direction":u16, "Trigger Delay (samples)":u32, "Auto Trigger Time (ms)":i16}}
  T3 = cluster{"Auto Stop":bool, "Desired Sample Interval":u32, "Pre-trigger Samples":u32, "Post-trigger Samples":u32, "Down-Sample Ratio":u32, "Down-Sample Mode":i32, "Overview Buffer Size":u32, "Time Units":u32}
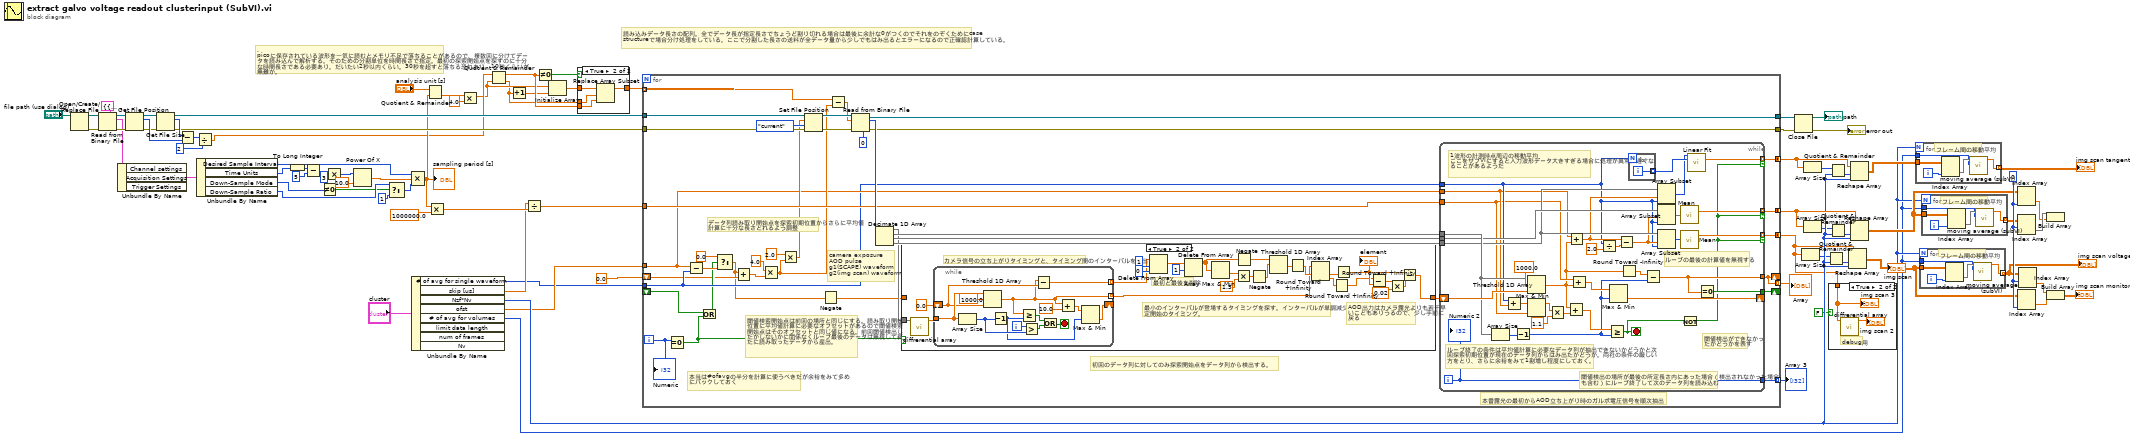
[diagram p0: block diagram]
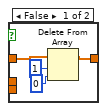
[diagram p3: hidden frame]
diagram:
  w76 = 0 ("disabled index (col) 2")
  # "読み込みデータ長さの配列。全でデータ長が指定長さでちょうど割り切れる場合は最後に余計な0がつくのでそれをのぞくためにcase structureで場合分け処理をしている。ここで分割した長さの送料が全データ量から少しでもはみ出るとエラーになるので正確認計算している。"
  # ".picoに保存されている波形を一気に読むとメモリ不足で落ちることがあるので、複数回に分けてデータを読み込んで解析する。そのための分割単位を時間長さで指定。最初の探索開始点を探すのに十分な時間長さである必要あり。だいたい2秒以内くらい。30秒を超すと落ちる恐れあり。10秒くらいが無難か。"
  n1 = Open/Create/Replace File(file path (use dialog)="file path (use dialog)") -> (refnum out=w39:refnum<file>, error out=w40:errorcluster)  [unwired: 5 in, 1 out]
  n2 = Read from Binary File(5:T2 {"Channel settings"={"Ch D  sync"={"Enabled"=FALSE, "Coupling"=0, "Range"=0, "Offset"=0.0}, "Ch C AWG "={"Enabled"=FALSE, "Coupling"=0, "Range"=0, "Offset"=0.0}, "Ch G scape"={"Enabled"=FALSE, "Coupling"=0, "Range"=0, " Offset"=0.0}, "Ch H img scan"={"Enabled"=FALSE, "Coupling"=0, "Range"=0, "Offset"=0.0}, "Ch B Cam"={"Enabled"=FALSE, "Coupling"=0, "Range"=0, "Offset"=0.0}, "Ch A"={"Enabled"=FALSE, "Coupling"=0, "Range"=0, "Offset"=0.0}, "Ch E"={"Enabled"=FALSE, "Coupling"=0, "Range"=0, "Offset"=0.0}, "Ch F"={"Enabled"=FALSE, "Coupling"=0, "Range"=0, "Offset"=0.0}}, "Acquisition Settings"={"Auto Stop"=FALSE, "Desired Sample Interval"=0, "Pre-trigger Samples"=0, "Post-trigger Samples"=0, "Down-Sample Ratio"=0, "Down-Sample Mode"=0, "Overview Buffer Size"=0, "Time Units"=0}, "Trigger Settings"={"Trigger Enabled"=FALSE, "Trigger Source"=enum."Channel A", "Trig Thresh (16-bit counts)"=0, "Trigger Direction"=0, "Trigger Delay (samples)"=0, "Auto Trigger Time (ms)"=0}} ("output cluster"), 8:w40, 11:w39) -> (0:w61:errorcluster, 2:w42:T2, 3:w59:refnum<file>)  [unwired: 3 in, 1 out]
  n3 = Unbundle By Name(w42) -> ("Acquisition Settings"=w43:T3)  [unwired: 2 out]
  n4 = Get File Position(4:w61, 7:w59) -> (0:w58:errorcluster, 2:w65:i64, 3:w60:refnum<file>)
  n5 = Get File Size(file=w60, error in=w58) -> (refnum out=w62:refnum<file>, size (in bytes)=w64:i64, 0:w63:errorcluster)
  n6 = Subtract(x=w64, y=w65) -> (x-y=w66:i64)
  n7 = Divide(x=w66, y=i64 2) -> (x/y=w25:dbl)
  n8 = Unbundle By Name(w43) -> ("Desired Sample Interval"=w50:u32, "Time Units"=w44:u32, "Down-Sample Mode"=w52:i32, "Down-Sample Ratio"=w54:u32)
  n9 = To Long Integer(number=w44) -> (32bit integer=w57:i32)
  n10 = Subtract(x=w57, y=5 ("x")) -> (x-y=w46:i32)
  n11 = Not Equal To 0?(x=w52) -> (x != 0?=w53:bool)
  n12 = Multiply(x=w46, y=3) -> (x*y=w49:i32)
  n13 = Power Of X(1:10.0 ("x"), 2:w49) -> (0:w51:dbl)
  n14 = Select(t=w54, s=w53, f=1) -> (s? t:f=w56:u32)
  n15 = Compound Arithmetic op=MULTIPLY(w50, w51, w56) -> (w26:dbl)
  "sampling period [s]" <- w26
  n16 = Unbundle By Name("cluster") -> ("# of avg for single waveform"=w6:u16, "skip [us]"=w34:dbl, "Nzf*Nv"=w37:i32, "ofst"=w7:dbl, "# of avg for volumes"=w36:u16)  [unwired: 3 out]
  n17 = Quotient & Remainder(x="analysis unit [s]", y=w26) -> (floor(x/y)=w15:dbl)  [unwired: 1 out]
  n18 = Multiply(x=w26, y=1000000.0) -> (x*y=w35:dbl)
  n19 = Multiply(x=w15, y=4.0) -> (x*y=w14:dbl)
  n20 = Quotient & Remainder(x=w25, y=w14) -> (x-y*floor(x/y)=w22:dbl, floor(x/y)=w11:dbl)
  n21 = Increment(x=w11) -> (x+1=w12:dbl)
  n22 = Divide(x=w34, y=w35) -> (x/y=w8:dbl)
  n23 = Not Equal To 0?(x=w22) -> (x != 0?=w21:bool)
  n24 = Initialize Array(w14, w12) -> (w24:dbl[])
  n25 = case shown="True" w21 {
    tunnel: w24 -> [w84 w88]
    tunnel: w11 -> [_ w87]
    tunnel: w22 -> [_ w86]
    tunnel: [w83 w85] -> w23
    frame False {
      n26 = Delete From Array(array=w84, length=1, index=0) -> (array with subset deleted=w83:dbl[])  [unwired: 1 out]
    }
    frame True {
      n27 = Replace Array Subset(array=w88, new element=w86, index=w87) -> (w85:dbl[])
    }
  }
  n28 = for {
    tunnel: [w104] -> w78 mode=concatenating
    tunnel: [w92] -> w3 mode=concatenating
    tunnel: [w127] -> w68 mode=concatenating
    tunnel: w63 -> [w115]
    tunnel: w62 -> [w116]
    tunnel: w7 -> [w101]
    tunnel: w6 -> [w97]
    tunnel: w8 -> [w119]
    tunnel: w23 -> [w107] mode=indexing
    shift-right: [w96] -> _
    shift-left: 0.0 -> [w90]
    tunnel: [w111] -> w17
    tunnel: [w110] -> w16
    tunnel: [w96] -> w5 mode=indexing
    shift-right: [w95] -> _
    shift-left: _ -> [w93]
    tunnel: [w91] -> w4 mode=indexing
    i -> [w118]
    # "本当は#ofavgの半分を計算に使うべきだが余裕をみて多めにバックしておく"
    # "閾値検索開始点は前回の場所と同じにする。読み取り開始位置に平均値計算に必要なオフセットがあるので閾値検索開始点はそのオフセットと同じ値になる。前回閾値検出したかしないかに関係なくループ最後のデータは無視して新たに読み取ったデータから産出。"
    # "初回のデータ列に対してのみ探索開始点をデータ列から検出する。"
    # "データ列読み取り開始点を探索初期位置からさらに平均値計算に十分な長さとれるよう調整"
    # "camera exposure\nAOD pulse\ng1(SCAPE) waveform\ng2(img scan) waveform"
    # "本番露光の最初からAOD立ち上がり時のガルボ電圧信号を順次抽出"
    n29 = Equal To 0?(x=w118) -> (x = 0?=w100:bool)
    n30 = Subtract(x=w101, y=w97) -> (x-y=w98:dbl)
    n31 = Or(x=w93, y=w100) -> (x .or. y?=w94:bool)
    n32 = Select(t=0.0, s=w94, f=w98) -> (s? t:f=w89:dbl)
    n33 = Add(x=w89, y=w90) -> (x+y=w103:dbl)
    n34 = Multiply(x=4.0, y=w103) -> (x*y=w105:dbl)
    n35 = Multiply(x=2.0, y=w105) -> (x*y=w106:dbl)
    n36 = Set File Position(offset (in bytes) (0)=w106, refnum=w116, from (0:start)=enum16{"start", "end", "current"}."current", error in=w115) -> (refnum out=w114:refnum<file>, error out=w113:errorcluster)
    n37 = Negate(x=w89) -> (-x=w102:dbl)
    n38 = Subtract(x=w107, y=w105) -> (x-y=w108:dbl)
    n39 = Read from Binary File(5:i16 0, 8:w113, 10:w108, 11:w114) -> (0:w111:errorcluster, 2:w126:i16[], 3:w110:refnum<file>)  [unwired: 2 in, 1 out]
    n40 = Decimate 1D Array(w126) -> (w120:i16[], w121:i16[], w123:i16[], w122:i16[])
    n41 = case shown="True" w100 {
      tunnel: [w128 w132] -> w124
      tunnel: w120 -> [_ w131]
      tunnel: w102 -> [w128 _]
      frame False {
      }
      frame True {
        # "AOD出力はカメラ露光よりも若干早いこともありうるので、少し手前に戻る"
        # "最小のインターバルが登場するタイミングを探す。インターバルが単調減少するので、そこが本番測定開始のタイミング。"
        # "最初と最後を削除"
        # "カメラ信号の立ち上がりタイミングと、タイミング間のインターバルを抽出"
        n42 = call "diffrerential array.vi"("Array in"=w131) -> ("Array"=w133:dbl[])  [unwired: 10 in]
        n43 = while {
          shift-right: [w156] -> _
          shift-left: 0.0 -> [w161]
          tunnel: w133 -> [w162]
          tunnel: [w158] -> w130 mode=indexing
          tunnel: [w160] -> w129 mode=indexing
          i -> [w164]
          stop <- w159 stop-if-true
          n44 = Array Size(array=w162) -> (size(s)=w163:i32)
          n45 = Threshold 1D Array(1:w161, 2:1000.0 ("threshold y"), 3:w162) -> (0:w158:dbl)
          n46 = Decrement(x=w163) -> (x-1=w154:i32)
          n47 = Greater Or Equal?(x=w158, y=w154) -> (x >= y?=w166:bool)
          n48 = Greater?(x=w164, y=w163) -> (0:w165:bool)
          n49 = Subtract(x=w158, y=w161) -> (x-y=w160:dbl)
          n50 = Or(x=w166, y=w165) -> (x .or. y?=w159:bool)
          n51 = Add(x=w158, y=10.0) -> (x+y=w155:dbl)
          n52 = Max & Min(x=w155, y=w154) -> (min(x,y)=w156:dbl)  [unwired: 1 out]
        }
        n53 = Delete From Array(array=w129, length=1, index=0) -> (array with subset deleted=w137:dbl[])  [unwired: 1 out]
        n54 = Delete From Array(array=w137, length=1) -> (array with subset deleted=w147:dbl[])  [unwired: 1 in, 1 out]
        n55 = Array Max & Min(array=w147) -> (min value=w139:dbl)  [unwired: 3 out]
        n56 = Multiply(x=w139, y=1.5) -> (x*y=w141:dbl)
        n57 = Negate(x=w147) -> (-x=w142:dbl[])
        n58 = Negate(x=w141) -> (-x=w143:dbl)
        n59 = Threshold 1D Array(2:w143, 3:w142) -> (0:w144:dbl)  [unwired: 1 in]
        n60 = Round Toward +Infinity(x=w144) -> (ceil(x): smallest int >= x=w145:dbl)
        n61 = Index Array(array=w130, index #1=w145) -> (element #1=w146:dbl, element #2=w148:dbl)  [unwired: 1 in]
        n62 = Round Toward +Infinity(x=w148) -> (ceil(x): smallest int >= x=w149:dbl)
        n63 = Round Toward +Infinity(x=w146) -> (ceil(x): smallest int >= x=w150:dbl)
        "element" <- w150
        n64 = Subtract(x=w149, y=w150) -> (x-y=w151:dbl)
        n65 = Multiply(x=w151, y=0.02) -> (x*y=w153:dbl)
        n66 = Subtract(x=w150, y=w153) -> (x-y=w132:dbl)
      }
    }
    n67 = while {
      tunnel: w121 -> [w200]
      shift-right: [w198] -> _
      shift-left: w124 -> [w201]
      tunnel: w123 -> [w196]
      tunnel: [w195] -> w127 mode=indexing if=w169
      tunnel: w122 -> [w190]
      tunnel: [w194] -> w92 mode=indexing if=w169
      tunnel: [w176] -> w104 mode=indexing if=w169
      tunnel: w97 -> [w184]
      tunnel: w101 -> [w183]
      tunnel: w119 -> [w181]
      tunnel: [w171] -> w96
      tunnel: [w170] -> w95
      tunnel: [w168] -> w91
      i -> [w168]
      stop <- w175 stop-if-true
      # "ループの最後の計算値を無視する"
      # "閾値検出ができなかったかどうかを表す"
      # "ループ終了の条件は平均値計算に必要なデータ列が抽出できないかどうかと次回探索初期位置が現在のデータ列からはみ出たかどうか。両社の条件の厳しい方をとり、さらに余裕をみて1割増し程度にしておく。"
      # "閾値検出の場所が最後の所定長さ内にあった場合（検出されなかった場合も含む）にループ終了して次のデータ列を読み込む"
      # "1波形の計測時点周辺の移動平均\nここをサブVIにすると入力波形データ大きすぎる場合に処理が異常に遅くなることがあるようだ"
      n68 = Array Size(array=w200) -> (size(s)=w199:i32)
      n69 = Add(x=w184, y=w183) -> (x+y=w182:dbl)
      n70 = Decrement(x=w199) -> (x-1=w173:i32)
      n71 = Max & Min(x=w182, y=w181) -> (max(x,y)=w180:dbl)  [unwired: 1 out]
      n72 = Threshold 1D Array(1:w201, 2:1000.0 ("threshold y"), 3:w200) -> (0:w174:dbl)
      n73 = Multiply(x=w180, y=1.1) -> (x*y=w178:dbl)
      n74 = Add(x=w174, y=w178) -> (x+y=w185:dbl)
      n75 = Add(x=w183, y=w174) -> (x+y=w187:dbl)
      n76 = Add(x=w181, y=w174) -> (x+y=w186:dbl)
      n77 = Divide(x=w184, y=2.0) -> (x/y=w188:dbl)
      n78 = Greater Or Equal?(x=w185, y=w173) -> (x >= y?=w175:bool)
      n79 = Max & Min(x=w186, y=w173) -> (min(x,y)=w198:dbl)  [unwired: 1 out]
      n80 = Subtract(x=w187, y=w188) -> (x-y=w189:dbl)
      n81 = Round Toward -Infinity(1:w174) -> (0:w172:dbl)
      n82 = for {
        N: w184 -> [_]
        tunnel: [w203] -> w192 mode=indexing
        i -> [w203]
      }
      n83 = Subtract(x=w172, y=w173) -> (x-y=w171:dbl)
      n84 = Array Subset(array=w196, index=w189, length=w184) -> (w193:i16[])
      n85 = Array Subset(array=w190, index=w189, length=w184) -> (w191:i16[])
      n86 = Array Subset(array=w190, index=w187, length=w184) -> (w177:i16[])
      n87 = call-poly <vilib>:"Mean.vi"("X"=w193) -> ("mean"=w195:dbl)  [unwired: 1 out]
      n88 = call-poly <vilib>:"Mean.vi"("X"=w191) -> ("mean"=w194:dbl)  [unwired: 1 out]
      n89 = Not(x=w175) -> (.not. x?=w169:bool)
      n90 = call <vilib>:"Linear Fit.vi"("Y"=w177, "X"=w192) -> ("slope"=w176:dbl)  [unwired: 9 in, 4 out]
      n91 = Equal To 0?(x=w171) -> (x = 0?=w170:bool)
      "Numeric 2" <- w168
    }
    "Numeric" <- w118
  }
  "Array" <- w5
  "Array 3" <- w4
  n92 = Close File(refnum=w16, error in=w17) -> (path=→"path":path, error out=→"error out":errorcluster)
  n93 = Array Size(array=w3) -> (size(s)=w31:i32)
  n94 = Array Size(array=w68) -> (size(s)=w28:i32)
  n95 = Array Size(array=w78) -> (size(s)=w33:i32)
  n96 = Quotient & Remainder(x=w31, y=w37) -> (floor(x/y)=w30:i32)  [unwired: 1 out]
  n97 = case shown="True" FALSE {
    tunnel: w3 -> [_ w204]
    frame False {
    }
    frame True {
      # "debug用"
      n98 = call "diffrerential array.vi"("Array in"=w204) -> ("Array"=→"img scan 2":dbl[])  [unwired: 10 in]
      "img scan 3" <- w204
    }
  }
  n99 = Quotient & Remainder(x=w28, y=w37) -> (floor(x/y)=w29:i32)  [unwired: 1 out]
  n100 = Quotient & Remainder(x=w33, y=w37) -> (floor(x/y)=w32:i32)  [unwired: 1 out]
  n101 = Reshape Array(w3, w30, w37) -> (w1:dbl[][])
  "img scan" <- w1
  n102 = Reshape Array(w68, w29, w37) -> (w75:dbl[][])
  n103 = Reshape Array(w78, w32, w37) -> (w79:dbl[][])
  n104 = for {
    N: w37 -> [_]
    tunnel: w79 -> [w210]
    tunnel: [w209] -> w10 mode=indexing
    tunnel: w36 -> [w206]
    i -> [w207]
    # "フレーム間の移動平均"
    n105 = Index Array(array=w210, index (col)=w207) -> (element=w208:dbl[])  [unwired: 1 in]
    n106 = call "moving average (subVI).vi"("average num"=w206, "Array in"=w208) -> ("Array out"=w209:dbl[])  [unwired: 9 in]
  }
  "img scan tangent" <- w10
  n107 = for {
    N: w37 -> [_]
    tunnel: w1 -> [w215]
    tunnel: [w214] -> w9 mode=indexing
    tunnel: w36 -> [w211]
    i -> [w212]
    # "フレーム間の移動平均"
    n108 = Index Array(array=w215, index (col)=w212) -> (element=w213:dbl[])  [unwired: 1 in]
    n109 = call "moving average (subVI).vi"("average num"=w211, "Array in"=w213) -> ("Array out"=w214:dbl[])  [unwired: 9 in]
  }
  "img scan voltage" <- w9
  n110 = for {
    N: w37 -> [_]
    tunnel: w75 -> [w220]
    tunnel: [w219] -> w74 mode=indexing
    tunnel: w36 -> [w216]
    i -> [w217]
    # "フレーム間の移動平均"
    n111 = Index Array(array=w220, index (col)=w217) -> (element=w218:dbl[])  [unwired: 1 in]
    n112 = call "moving average (subVI).vi"("average num"=w216, "Array in"=w218) -> ("Array out"=w219:dbl[])  [unwired: 9 in]
  }
  n113 = Index Array(array=w75, index (col)=w76) -> (element=w72:dbl[])  [unwired: 1 in]
  n114 = Index Array(array=w74, index (row)=w76) -> (element=w73:dbl[])  [unwired: 1 in]
  n115 = Index Array(array=w1, index (col)=w76) -> (element=w71:dbl[])  [unwired: 1 in]
  n116 = Index Array(array=w9, index (row)=w76) -> (element=w70:dbl[])  [unwired: 1 in]
  n117 = Build Array(w73, w72) -> ()  [unwired: 1 out]
  n118 = Build Array(w70, w71) -> (→"img scan monitor":dbl[][])
